vi "Main.vi"() -> ()   [LabVIEW 2018] (continued)
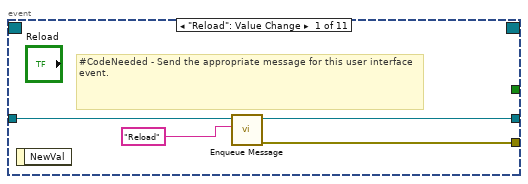
[diagram p3: hidden frame]
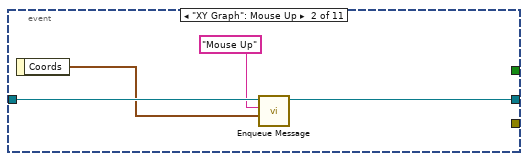
[diagram p4: hidden frame]
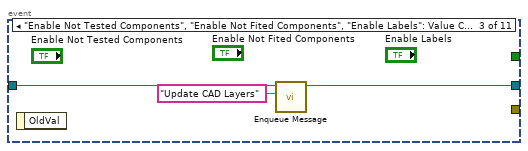
[diagram p5: hidden frame]
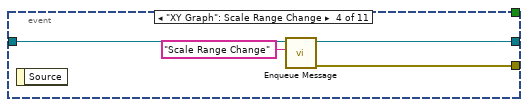
[diagram p6: hidden frame]
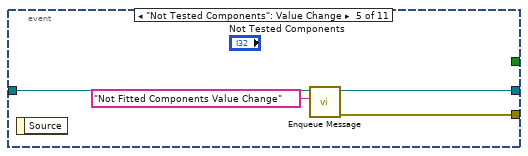
[diagram p7: hidden frame]
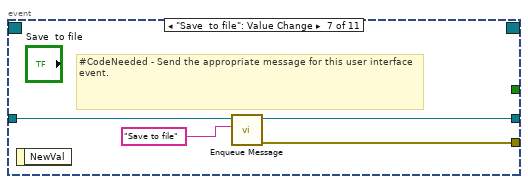
[diagram p8: hidden frame]
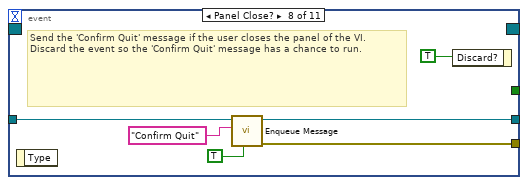
[diagram p9: hidden frame]
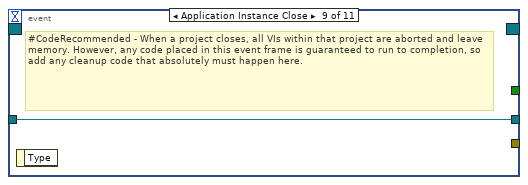
[diagram p10: hidden frame]
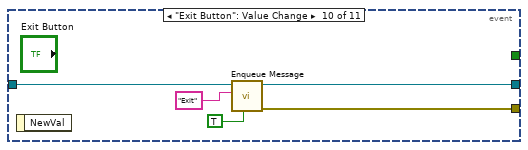
[diagram p11: hidden frame]
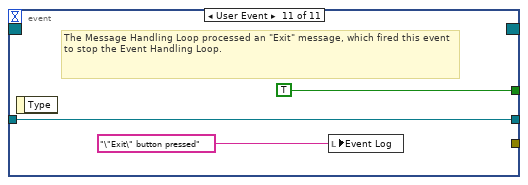
[diagram p12: hidden frame]
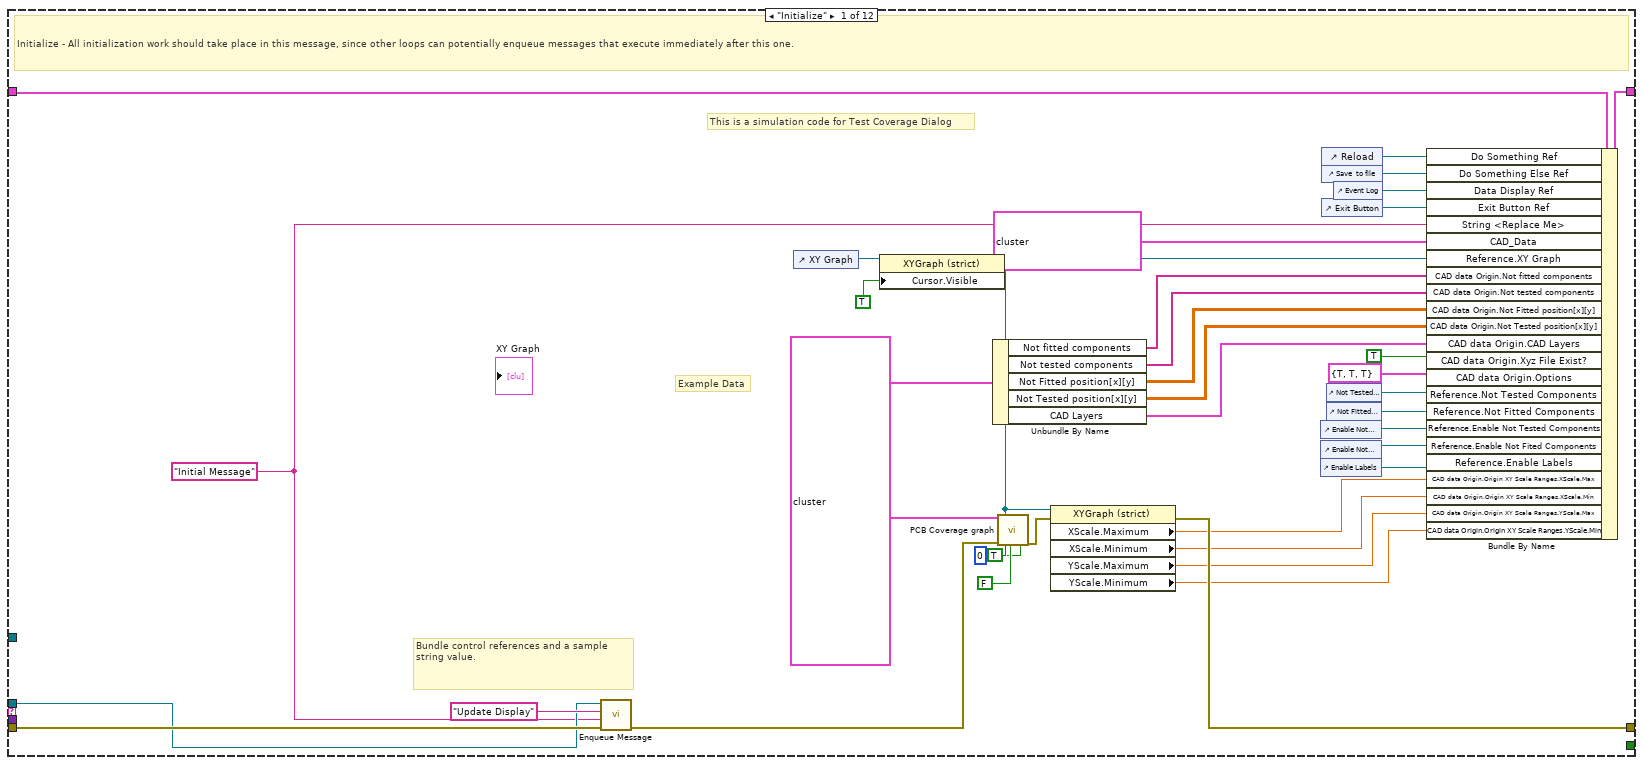
[diagram p13: hidden frame]
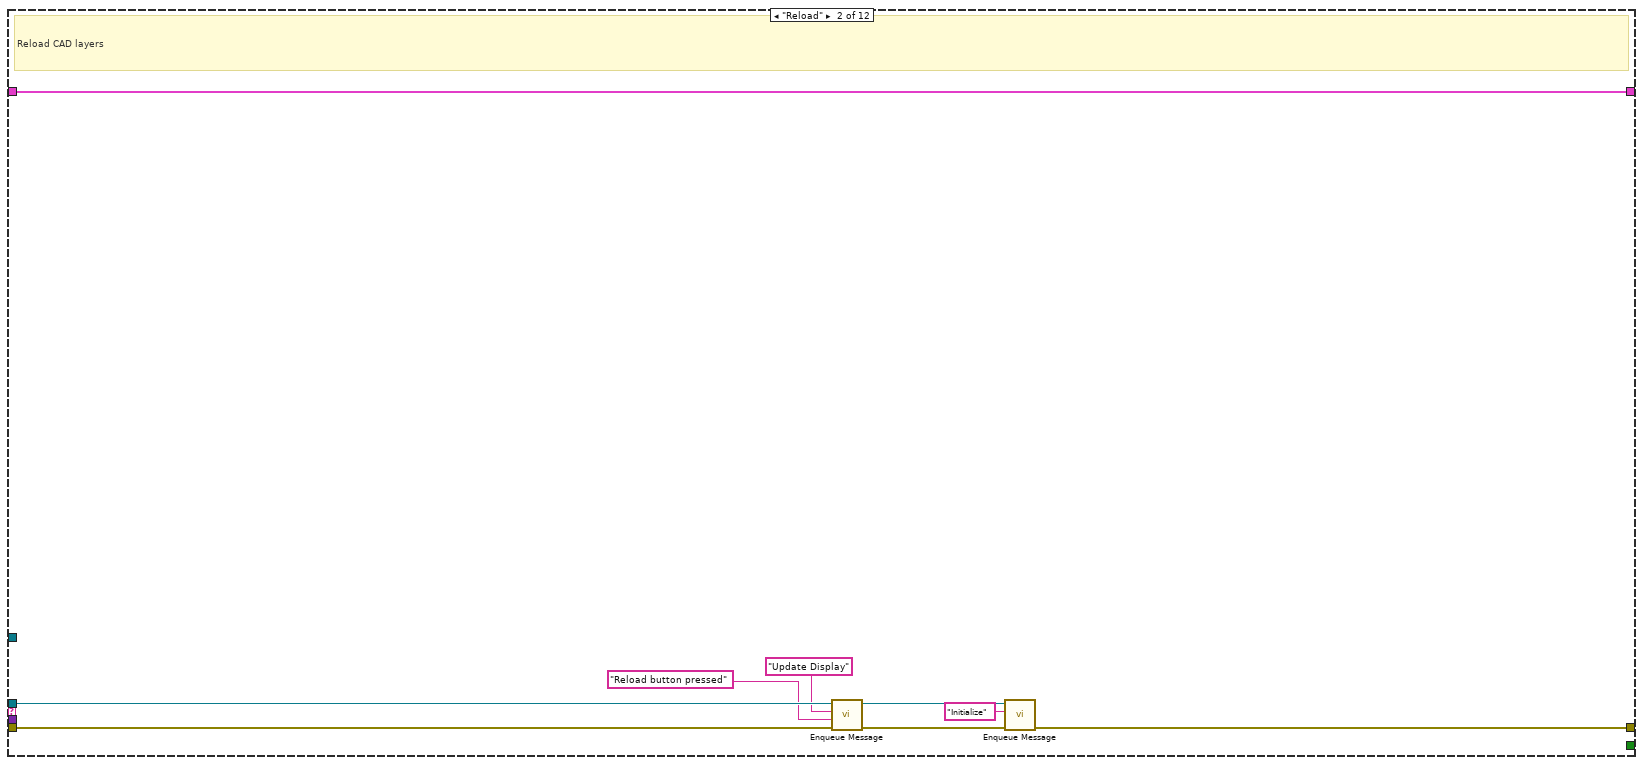
[diagram p14: hidden frame]
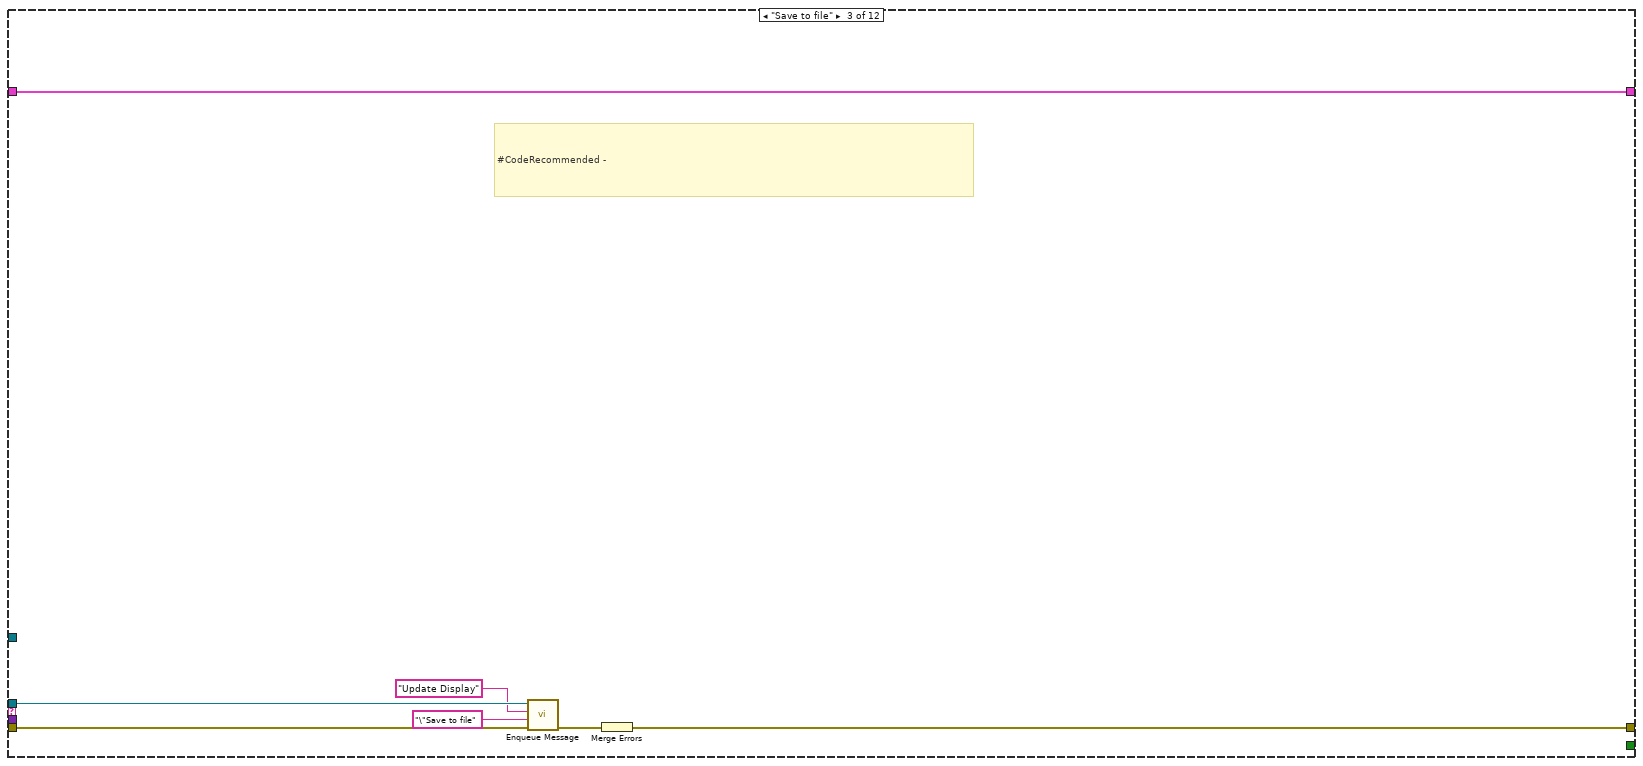
[diagram p15: hidden frame]
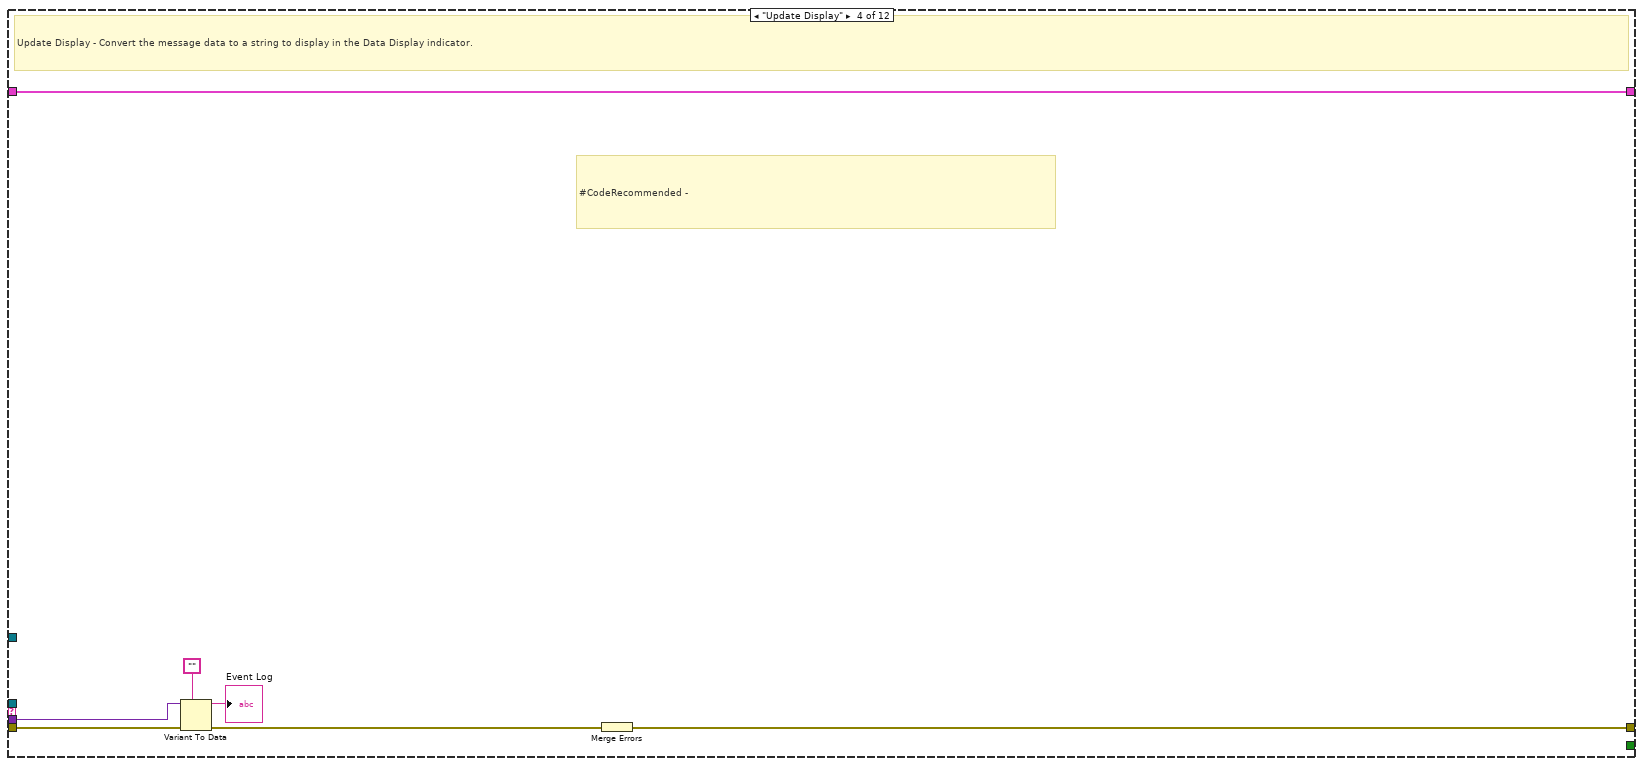
[diagram p16: hidden frame]
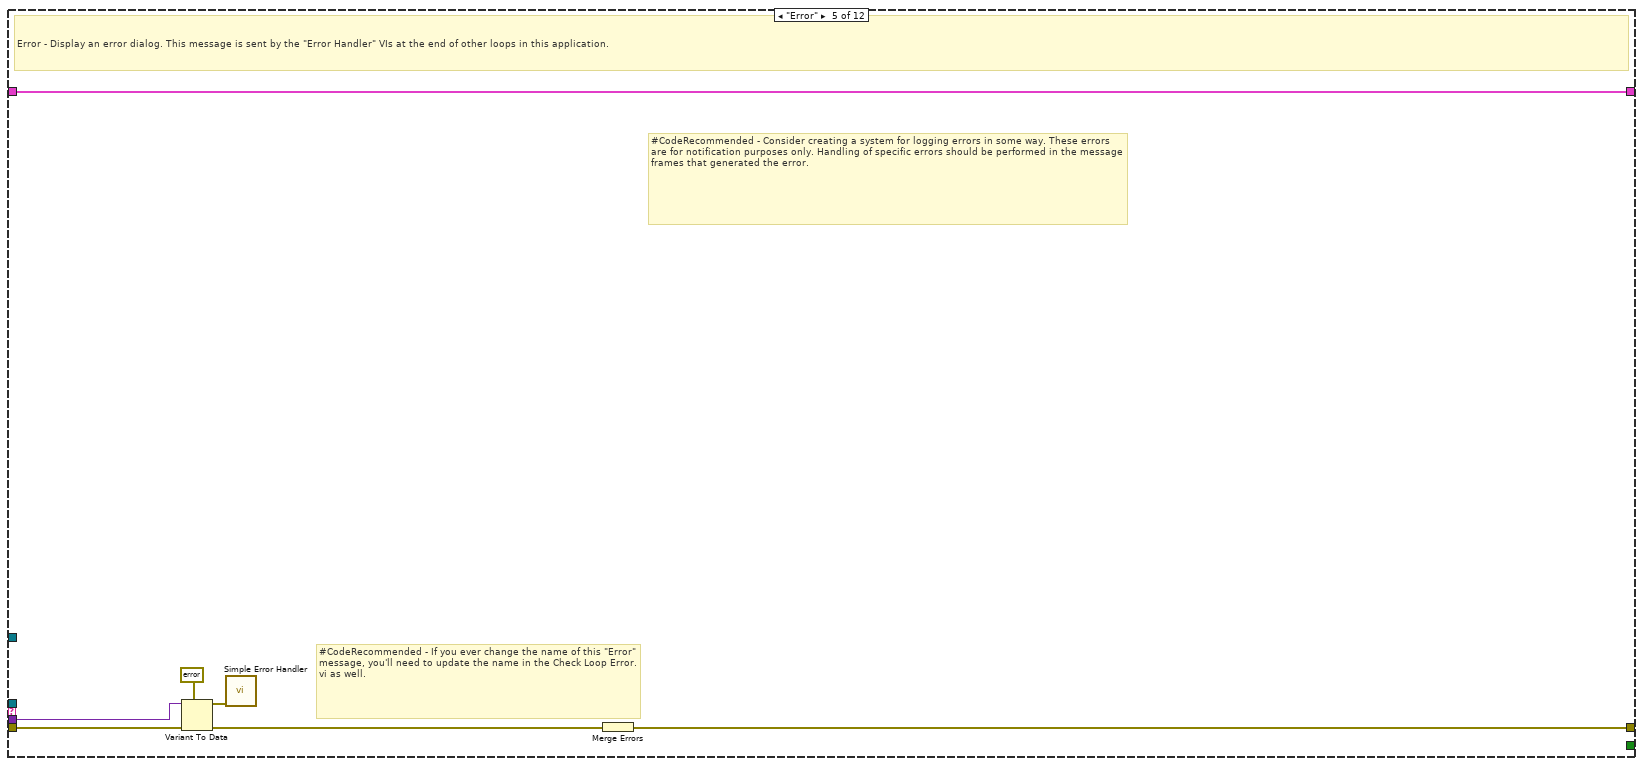
[diagram p17: hidden frame]
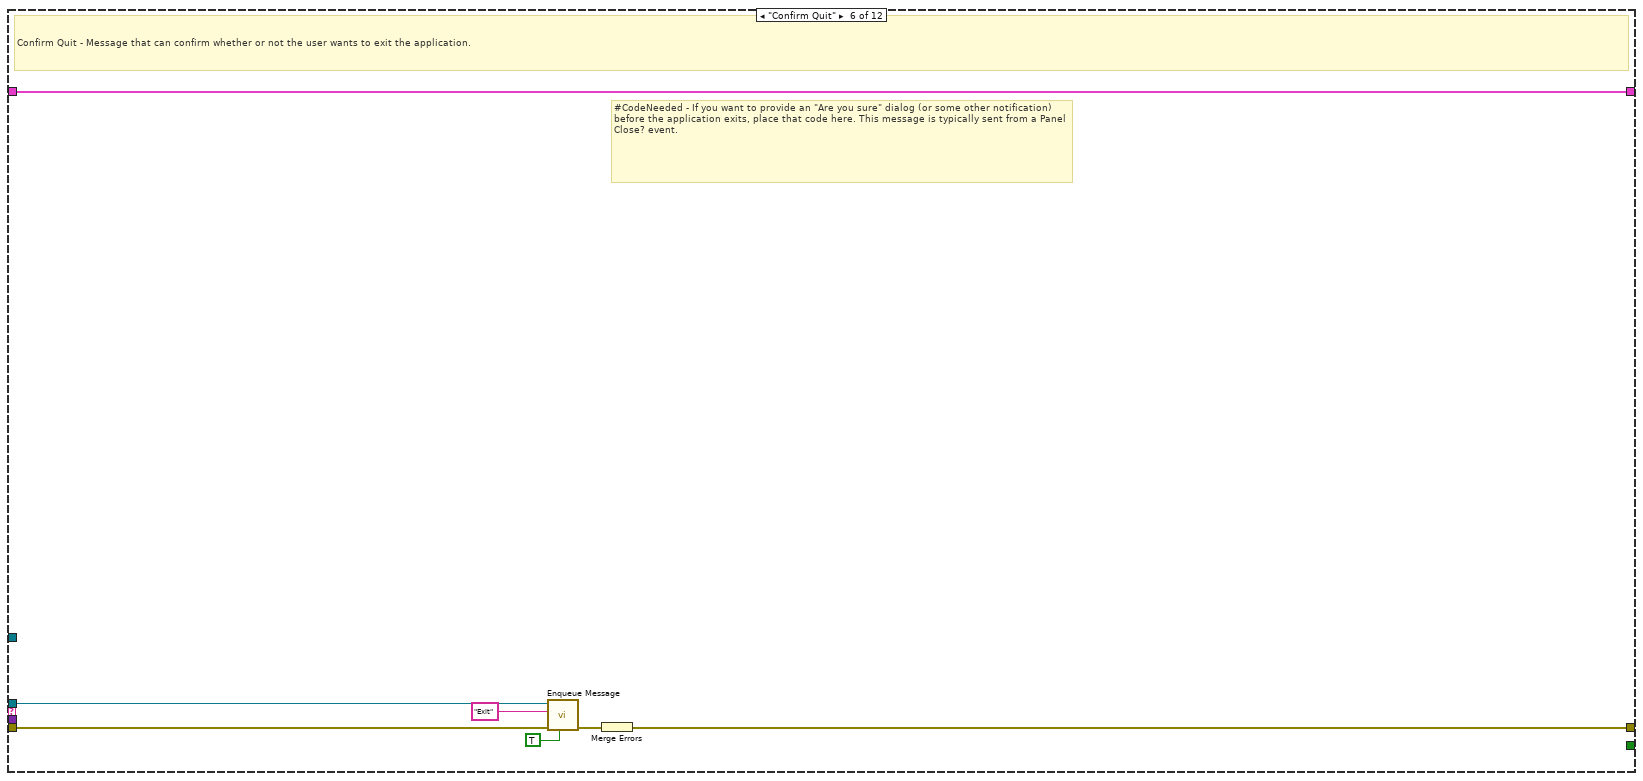
[diagram p18: hidden frame]
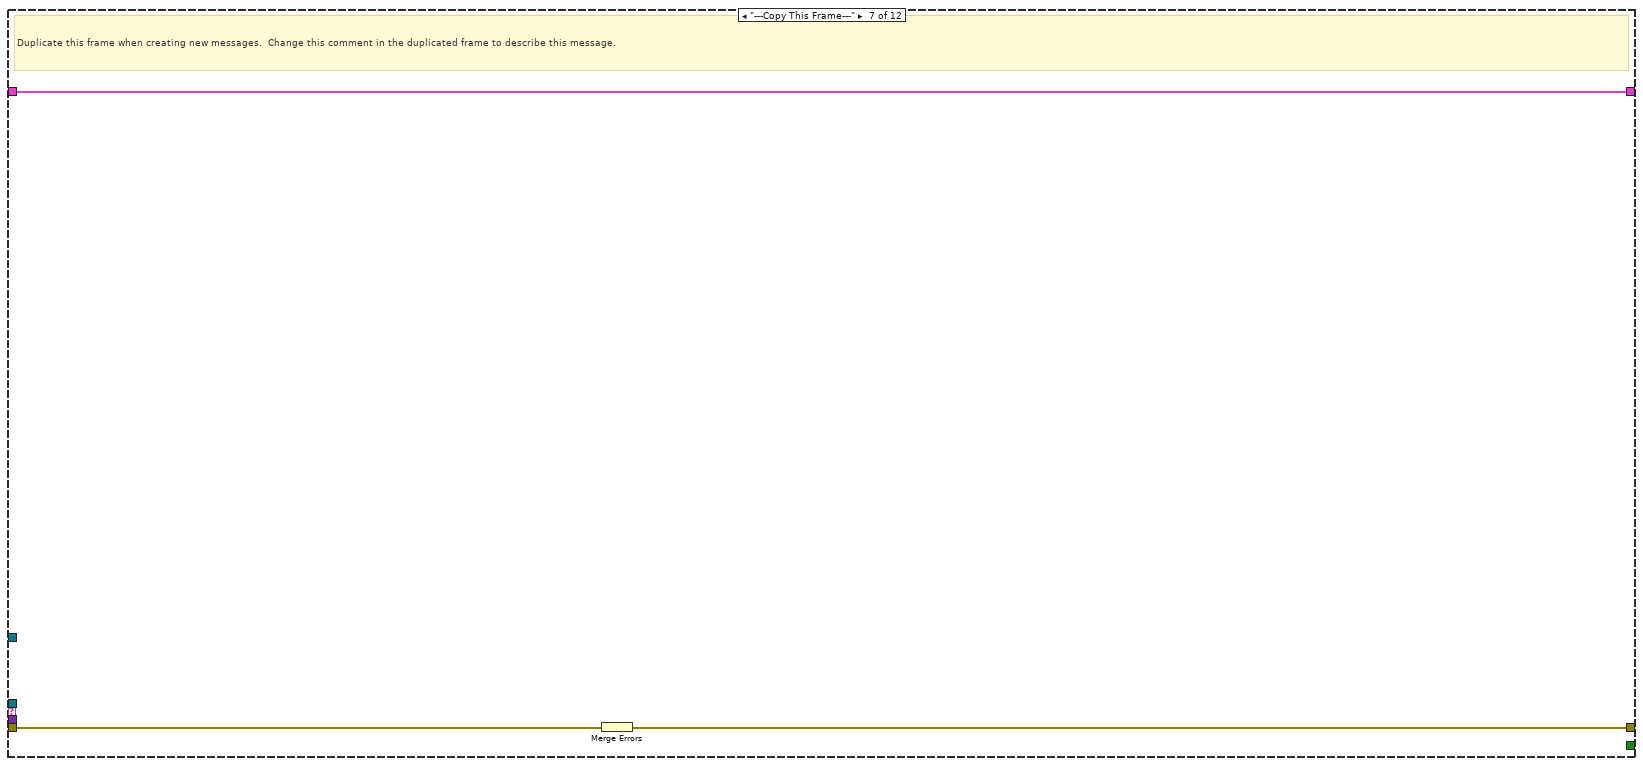
[diagram p19: hidden frame]
        n114 = Variant To Data(type=T3 {"Horizontal"=0, "Vertical"=0} ("Coords"), Variant=w318) -> (data=w277:T3)  [unwired: 1 in, 1 out]
        n115 = Unbundle By Name(w319) -> ("Reference.Not Tested Components"=w279:refnum<vi>, "Reference.Not Fitted Components"=w280:refnum<vi>, "CAD data Origin.Not tested components"=w287:string[], "CAD data Origin.Not fitted components"=w288:string[], "CAD data Origin.Not Tested position[x][y]"=w284:dbl[][], "CAD data Origin.Not Fitted position[x][y]"=w283:dbl[][], "Reference.XY Graph"=w281:refnum<vi>)
        n116 = invoke class="XYGraph (strict)" method="Map Coords To XY"(reference=w281, "Coords"=w277) -> (reference out=w290:refnum<vi>, error out=w289:errorcluster, "XY"=w286:cluster{"X":dbl, "Y":dbl})  [unwired: 5 in, 4 out]
        n117 = property on="Property Node" class="XYGraph (strict)"(reference=w290, error in=w289, "Cursor.Cursor Position"=w286) -> (reference out=w293:refnum<vi>, error out=w294:errorcluster, "Cursor.Cursor Position"=w276:T5, "XScale.Offset"=w317:dbl, "YScale.Offset"=w316:dbl, "XScale.Multiplier"=w315:dbl, "YScale.Multiplier"=w314:dbl)
        n118 = Build Array (concatenate)(w284, w283) -> (w303:dbl[][])
        n119 = Array Size(array=w284) -> (size(s)=w305:i32[])
        n120 = Build Array (concatenate)(w287, w288) -> (w298:string[])
        n121 = Index Array(array=w305) -> (element=w302:i32)  [unwired: 1 in]
        n122 = Index Array(array=w303, index (col) #1=0 ("disabled index (col)")) -> (element #1=w307:dbl[], element #2=w306:dbl[])  [unwired: 3 in]
        n123 = for {
          tunnel: w306 -> [w358] mode=indexing
          tunnel: w307 -> [w359] mode=indexing
          tunnel: [w357] -> w309 mode=indexing
          n124 = Bundle("String"=w359, "String"=w358) -> (w357:cluster{"String":dbl, "String":dbl})  [unwired: 1 in]
        }
        n125 = Bundle("XScale.Offset"=w317, "YScale.Offset"=w316) -> (w312:T10)  [unwired: 1 in]
        n126 = Bundle("XScale.Multiplier"=w315, "YScale.Multiplier"=w314) -> (w285:T11)  [unwired: 1 in]
        n127 = Subtract(x=w276, y=w312) -> (x-y=w313:T5)
        n128 = Merge Errors(w321) -> (w320:errorcluster)
        n129 = Divide(x=w313, y=w285) -> (x/y=w301:T5)
        n130 = property on="Property Node" class="XYGraph (strict)" props=["AnntList"](reference=w293, error in=w294) -> (reference out=w291:refnum<vi>, error out=w292:errorcluster)  [unwired: 1 out]
        n131 = Subtract(x=w309, y=w301) -> (x-y=w310:T5[])
        n132 = Re/Im To Polar(2:w301, 3:w310) -> (1:w311:T5[])  [unwired: 1 out]
        n133 = Array Max & Min(array=w311) -> (min index (indices)=w273:i32)  [unwired: 3 out]
        n134 = Index Array(array=w298, index=w273) -> (element=w297:string)
        n135 = Greater?(x=w302, y=w273) -> (0:w304:bool)
        n136 = Unbundle(w301) -> ("Cursor X"=w299:dbl, "Cursor Y"=w300:dbl)
        n137 = Format Into String(format string="%s  (%.3fmm,%.3fmm)", w297, w299, w300) -> (resulting string=w295:string)  [unwired: 2 in, 1 out]
        n138 = case shown="True" w304 {
          tunnel: w292 -> [w331 w347]
          tunnel: w273 -> [w335 w350]
          tunnel: [w341 w349] -> w278
          tunnel: w302 -> [w333 _]
          tunnel: w280 -> [w329 w345]
          tunnel: w279 -> [w327 w344]
          frame False {
            n139 = property on="Property Node" class="LstBox (strict)"(reference=w327, error in=w331, "Value"=-1 ("Not Tested Components")) -> (error out=w330:errorcluster)  [unwired: 1 out]
            n140 = Subtract(x=w335, y=w333) -> (x-y=w334:i32)
            n141 = property on="Property Node" class="LstBox (strict)"(reference=w329, error in=w330) -> (reference out=w328:refnum<vi>, error out=w342:errorcluster, "Number of Rows"=w337:u32, "Top Row"=w336:i32)
            n142 = Add(x=w337, y=w336) -> (x+y=w339:u32)
            n143 = In Range and Coerce(upper limit=w339, x=w334, lower limit=w336) -> (In Range?=w340:bool)  [unwired: 1 out]
            n144 = Select(t=w336, s=w340, f=w334) -> (s? t:f=w338:i32)
            n145 = property on="Property Node" class="LstBox (strict)"(reference=w328, error in=w342, "Value"=w334, "Top Row"=w338) -> (error out=w341:errorcluster)  [unwired: 1 out]
          }
          frame True {
            n146 = property on="Property Node" class="LstBox (strict)"(reference=w345, error in=w347, "Value"=-1 ("Not Tested Components")) -> (error out=w346:errorcluster)  [unwired: 1 out]
            n147 = property on="Property Node" class="LstBox (strict)"(reference=w344, error in=w346) -> (reference out=w343:refnum<vi>, error out=w356:errorcluster, "Number of Rows"=w353:u32, "Top Row"=w352:i32)
            n148 = Add(x=w353, y=w352) -> (x+y=w354:u32)
            n149 = In Range and Coerce(upper limit=w354, x=w350, lower limit=w352) -> (In Range?=w355:bool)  [unwired: 1 out]
            n150 = Select(t=w352, s=w355, f=w350) -> (s? t:f=w351:i32)
            n151 = property on="Property Node" class="LstBox (strict)"(reference=w343, error in=w356, "Value"=w350, "Top Row"=w351) -> (error out=w349:errorcluster)  [unwired: 1 out]
          }
        }
        n152 = Bundle By Name(cluster=T6 {"Name"="", "Color"=0, "Style"=0, "Point Style"=0, "Name Visible"=FALSE, "Allow Drag"=FALSE, "Annotation Mode"=0, "Plot"=0, "Index"=0, "Position"={"X"=0.0, "Y"=0.0}, "X Scale"=0, "Y Scale"=0, "Show Arrow"=FALSE, "Lock Name"=FALSE, "Plot Area"=0, "Label Offset"={"X"=0.0, "Y"=0.0}} ("element"), "Label Offset"=cluster{"X":dbl, "Y":dbl} {"X"=1.0, "Y"=1.0}, "Color"=u32 16448250, "Show Arrow"=w272, "Name Visible"=w272, "Name"=w295, "Index"=w273, "Position"=w276) -> (w275:T6)
        n153 = disable-structure shown="Disabled" {
          disable-tunnel: w275 -> [w325 w326]
          disable-tunnel: [w324 w326] -> w269
          disable-tunnel: w276 -> [w322 _]
          frame Disabled {
            n154 = call "Fid graph annotation label offset.vi"("Annotation List"=w325, "Load Graph Centre x, y"=FALSE, "Cursor Position"=w322) -> ("Annotation List"=w324:T6)  [unwired: 12 in]
          }
          frame Enabled {
          }
        }
        n155 = Build Array(w269) -> (w268:T12)
        n156 = property on="Property Node" class="XYGraph (strict)" props=["AnntList", "Cursor"](reference=w291, error in=w278, "AnntList"=w268) -> ()  [unwired: 3 out]
      }
      frame "Exit" {
        # "Stop the VI"
        # "Release the message queue reference"
        # "#CodeNeeded - Add any required cleanup code here. Note that if 'Exit' was called as a result of an error, an error dialog will be displayed. Add any custom error handling for an 'Exit' condition here as well."
        # "Exit - Exit the application."
        n157 = Variant To Data(type=errorcluster {"status"=FALSE, "code"=0, "source"=""} ("error constant"), Variant=w360) -> (data=w361:errorcluster)  [unwired: 1 in, 1 out]
        n158 = call <vilib>:"Simple Error Handler.vi"("error in (no error)"=w361) -> ()  [unwired: 4 in, 5 out]
        n159 = call "Fire User Event - Stop.vi"("User Event - Stop"=w365) -> ("error out"=w364:errorcluster)  [unwired: 10 in]
        n160 = Release Queue(queue=w370, error in (no error)=w363) -> (error out=w367:errorcluster)  [unwired: 1 in, 2 out]
        n161 = Merge Errors(w364, w367) -> (w366:errorcluster)
      }
      frame Default {
        # "'Default' case only runs if there is a message that isn't defined in any of the other cases.  Output a programming error."
        n162 = xnode "Error Ring"("parameter 0"=w371) -> ("error out"=w372:errorcluster)
      }
    }
    n163 = call "Error Handler - Message Handling Loop.vi"("error in (no error)"=w65, "Message Queue"=w67) -> ("dup error in"=w66:errorcluster)  [unwired: 8 in, 1 out]
  }
  n164 = Unregister For Events(event registration refnum=w8, error in=w5) -> (error out=w9:errorcluster)
  n165 = Merge Errors(w9, w13) -> (w10:errorcluster)
  n166 = call "Destroy User Event - Stop.vi"("error in (no error)"=w10, "User Event - Stop"=w3) -> ("error out"=w6:errorcluster)  [unwired: 9 in]
  n167 = disable-structure shown="RUN_TIME_ENGINE==True" {
    disable-tunnel: w6 -> [_ _]
    frame condition #0 (active) {
    }
    frame condition #1 {
      # "Call Quit LabVIEW if running as a built application."
      n168 = Quit LabVIEW() -> ()  [unwired: 1 in]
    }
  }
